vi "UHR-Fleezers Control (host) - 12.0.vi"() -> ()   [LabVIEW 2014] (continued)
            n2110 = property on="Trap Pos. FB ON" class="Bool (strict)"("Val(Sgnl)"=TRUE ("Value (Signaling)")) -> ()  [unwired: 2 in, 2 out]
            n2111 = Wait (ms)(milliseconds to wait=u32 250) -> ()  [unwired: 1 out]
          }
          frame #5 {
            n2112 = case shown="\"1\"" "Remove Action Offset Dropdown" {
              tunnel: TRUE ("Value (Signaling)") -> [w3020 w3028 w3036]
              frame "1" {
                n2113 = flat-sequence {
                  tunnel: w3020 -> [w3027]
                  frame #0 {
                    n2114 = local read "factor"() -> (w3022:dbl)
                    n2115 = Greater Than 0?(x=w3022) -> (x > 0?=w3026:bool)
                    n2116 = Select(t=1.0, s=w3026, f=-1.0) -> (s? t:f=w3023:dbl)
                    n2117 = Multiply(x=w3023, y=w3022) -> (x*y=w3021:dbl)
                    n2118 = local write "factor"(w3021) -> ()
                  }
                  frame #1 {
                    n2119 = property on="Remove Offset to factor" class="Bool (strict)"("Val(Sgnl)"=w3027) -> ()  [unwired: 2 in, 2 out]
                  }
                }
              }
              frame "2" {
                n2120 = flat-sequence {
                  tunnel: w3028 -> [w3035]
                  frame #0 {
                    n2121 = local read "factor"() -> (w3029:dbl)
                    n2122 = Greater Than 0?(x=w3029) -> (x > 0?=w3034:bool)
                    n2123 = Select(t=-1.0, s=w3034, f=1.0) -> (s? t:f=w3032:dbl)
                    n2124 = Multiply(x=w3029, y=w3032) -> (x*y=w3031:dbl)
                    n2125 = local write "factor"(w3031) -> ()
                  }
                  frame #1 {
                    n2126 = property on="Remove Offset to factor" class="Bool (strict)"("Val(Sgnl)"=w3035) -> ()  [unwired: 2 in, 2 out]
                  }
                }
              }
              frame "0", Default {
                n2127 = property on="Remove Action Offset" class="Bool (strict)"("Val(Sgnl)"=w3036) -> ()  [unwired: 2 in, 2 out]
              }
            }
            n2128 = case shown="False" "Trap Trig Fl." {
              frame False {
                n2129 = case shown="True" "Green ON after FB ON?" {
                  selector: "Green ON after FB ON?" -> [_ w3038]
                  frame False {
                  }
                  frame True {
                    n2130 = property on="Green ON/Interlacing" class="Bool (strict)"("Val(Sgnl)"=w3038) -> ()  [unwired: 2 in, 2 out]
                  }
                }
              }
              frame True {
              }
            }
            n2131 = Wait (ms)(milliseconds to wait=u32 250) -> ()  [unwired: 1 out]
          }
          frame #6 {
            n2132 = property on="Start Saving" class="Bool (strict)"("Val(Sgnl)"=TRUE ("Value (Signaling)")) -> ()  [unwired: 2 in, 2 out]
            n2133 = Wait (ms)(milliseconds to wait=u32 5000) -> ()  [unwired: 1 out]
          }
          frame #7 {
            w3042 = TRUE ("Value (Signaling)")
            n2134 = property on="Rem fb disp offset" class="Bool (strict)"("Val(Sgnl)"=w3042) -> ()  [unwired: 2 in, 2 out]
            n2135 = property on="Remove Offset" class="Bool (strict)"("Val(Sgnl)"=w3042) -> ()  [unwired: 2 in, 2 out]
            n2136 = Wait (ms)(milliseconds to wait=u32 100) -> ()  [unwired: 1 out]
          }
          frame #8 {
            n2137 = case shown="True" w3045 {
              frame False {
              }
              frame True {
                n2138 = local write "Trap Trig. Fl."(TRUE ("Value (Signaling)")) -> ()
              }
            }
          }
          frame #9 {
            n2139 = local read "Tether"() -> (w3048:bool)
            n2140 = And(x="Start dipping after?", y=w3048) -> (x .and. y?=w3047:bool)
            n2141 = case shown="True" w3047 {
              frame False {
              }
              frame True {
                n2142 = flat-sequence {
                  frame #0 {
                    n2143 = Multiply(x="Delay before dipping (s)", y=1000.0) -> (x*y=w3051:dbl)
                    n2144 = Wait (ms)(milliseconds to wait=w3051) -> ()  [unwired: 1 out]
                  }
                  frame #1 {
                    n2145 = property on="Dip for Protein" class="Bool (strict)"("Val(Sgnl)"=TRUE ("Value (Signaling)")) -> ()  [unwired: 2 in, 2 out]
                    n2146 = local write "Scripts"(T35."Dipping") -> ()
                  }
                }
              }
            }
          }
        }
      }
      event "Rupture Script": Value Change {
        n2147 = event-data() -> ()  [unwired: 1 in, 5 out]
        n2148 = local write "Rupture Script"(FALSE ("Rupture Script")) -> ()
        n2149 = flat-sequence {
          frame #0 {
            w3057 = TRUE
            w3062 = FALSE
            # "Number 6 for now is the\nrupture-experiment\nparameters."
            n2150 = local read "Starting Trap D (MHz)"() -> (w3063:dbl)
            n2151 = local write "Restart DMA? (AOD)"(w3062) -> ()
            n2152 = Replace Array Subset(array=u32[] [0] ("Index Values"), new element=6, index=0) -> (w3058:u32[])
            n2153 = local write "Save scans"(w3062) -> ()
            n2154 = property on="Trap D (MHz)" class="DigNum (strict)"("Val(Sgnl)"=w3063) -> ()  [unwired: 2 in, 2 out]
            n2155 = property on="Saved AOD Raster Scan Parameter Sets" class="Arr (strict)"("Index Values"=w3058) -> ()  [unwired: 2 in, 2 out]
            n2156 = property on="Start Saving" class="Bool (strict)"("Val(Sgnl)"=w3057) -> ()  [unwired: 2 in, 2 out]
            n2157 = property on="Green ON/Interlacing" class="Bool (strict)"("Val(Sgnl)"=w3057) -> ()  [unwired: 2 in, 2 out]
          }
          frame #1 {
            n2158 = property on="Load parameters" class="Bool (strict)"("Val(Sgnl)"=TRUE ("Value (Signaling)")) -> ()  [unwired: 2 in, 2 out]
          }
        }
      }
      event "Fixed Traps Script": Value Change {
        n2159 = event-data() -> ()  [unwired: 1 in, 5 out]
        n2160 = local write "Fixed Traps Script"(FALSE ("Fixed Traps Data\nScript")) -> ()
        n2161 = flat-sequence {
          frame #0 {
            n2162 = case shown="True" "Green ON" {
              frame False {
              }
              frame True {
                n2163 = property on="Green ON/Interlacing" class="Bool (strict)"("Val(Sgnl)"=TRUE) -> ()  [unwired: 2 in, 2 out]
              }
            }
            n2164 = local write "Offset (nm)"(0.0 ("Offset (nm)")) -> ()
            n2165 = property on="Sample Channel\nFlow" class="Bool (strict)"("Val(Sgnl)"=FALSE ("Value (Signaling)")) -> ()  [unwired: 2 in, 2 out]
            n2166 = property on="Trap D (MHz)" class="DigNum (strict)"("Val(Sgnl)"="Fixed Traps Trap Delta (MHz)") -> ()  [unwired: 2 in, 2 out]
          }
          frame #1 {
            n2167 = Wait (ms)(milliseconds to wait=u32 1000) -> ()  [unwired: 1 out]
          }
          frame #2 {
            n2168 = local write "Start Saving"(TRUE ("Start Saving")) -> ()
          }
          frame #3 {
            n2169 = local read "Bead Sep. Int. Time (s)"() -> (w3073:dbl)
            n2170 = Multiply(x=w3073, y=1000.0) -> (x*y=w3075:dbl)
            n2171 = Wait (ms)(milliseconds to wait=w3075) -> ()  [unwired: 1 out]
          }
          frame #4 {
            n2172 = property on="Remove Offset" class="Bool (strict)"("Val(Sgnl)"=TRUE ("Value (Signaling)")) -> ()  [unwired: 2 in, 2 out]
          }
          frame #5 {
            n2173 = property on="Dip for Protein" class="Bool (strict)"("Val(Sgnl)"="Start dipping after?") -> ()  [unwired: 2 in, 2 out]
          }
        }
      }
      event "Got DNA bead": Value Change {
        n2174 = event-data() -> ()  [unwired: 1 in, 5 out]
        n2175 = flat-sequence {
          frame #0 {
            w3079 = FALSE ("Key Focus")
            n2176 = local read "Daq spot flow on"() -> (w3080:bool)
            n2177 = case shown="True" w3080 {
              frame False {
              }
              frame True {
                n2178 = property on="Sample Channel\nFlow" class="Bool (strict)"("Val(Sgnl)"=TRUE ("Value (Signaling)")) -> ()  [unwired: 2 in, 2 out]
              }
            }
            n2179 = local write "Got DNA bead"(w3079) -> ()
            n2180 = property on="Got DNA bead" class="Bool (strict)"("Key Focus"=w3079) -> ()  [unwired: 2 in, 2 out]
          }
          frame #1 {
            n2181 = property on="Inject Pump 1" class="Bool (strict)"("Val(Sgnl)"=FALSE ("Value (Signaling)")) -> ()  [unwired: 2 in, 2 out]
          }
          frame #2 {
            n2182 = property on="Cal/Data Acq. Spot" class="Bool (strict)"("Val(Sgnl)"=TRUE ("Value (Signaling)")) -> ()  [unwired: 2 in, 2 out]
          }
        }
      }
      event "Take Stepping Data": Value Change {
        n2183 = event-data() -> ()  [unwired: 1 in, 5 out]
        n2184 = local read "Save ave N"() -> (w3092:dbl)
        n2185 = flat-sequence {
          tunnel: w3092 -> [w3094]
          tunnel: [w3094] -> w3087
          tunnel: [w3096] -> w3088
          tunnel: w3087 -> [w3096]
          tunnel: [w3098] -> w3089
          tunnel: w3088 -> [w3098]
          tunnel: [w3101] -> w3090
          tunnel: w3089 -> [w3101]
          tunnel: [w3103] -> w3091
          tunnel: w3090 -> [w3103]
          tunnel: [w3105] -> w3085
          tunnel: w3091 -> [w3105]
          tunnel: w3085 -> [w3108]
          tunnel: [w3108] -> w3084
          tunnel: w3084 -> [w3109]
          tunnel: [w3109] -> w3086
          tunnel: w3086 -> [w3115]
          frame #0 {
            n2186 = property on="Save ave N" class="DigNum (strict)"("Val(Sgnl)"="Save ave factor") -> ()  [unwired: 2 in, 2 out]
          }
          frame #1 {
            n2187 = Wait (ms)(milliseconds to wait=u32 100) -> ()  [unwired: 1 out]
          }
          frame #2 {
            n2188 = local read "Offset 2 Start (MHz)"() -> (w3100:dbl)
            n2189 = property on="Saved AOD Raster Scan Parameter Sets" class="Arr (strict)"("Index Values"=u32[] [2]) -> ()  [unwired: 2 in, 2 out]
            n2190 = property on="Trap D (MHz)" class="DigNum (strict)"("Val(Sgnl)"=w3100) -> ()  [unwired: 2 in, 2 out]
          }
          frame #3 {
            n2191 = property on="Load parameters" class="Bool (strict)"("Val(Sgnl)"=TRUE ("Value (Signaling)")) -> ()  [unwired: 2 in, 2 out]
          }
          frame #4 {
            n2192 = Wait (ms)(milliseconds to wait=u32 100) -> ()  [unwired: 1 out]
          }
          frame #5 {
            n2193 = property on="Trap Raster Scan" class="Bool (strict)"("Val(Sgnl)"=TRUE ("Value (Signaling)")) -> ()  [unwired: 2 in, 2 out]
          }
          frame #6 {
            n2194 = Wait (ms)(milliseconds to wait=u32 1000) -> ()  [unwired: 1 out]
          }
          frame #7 {
            n2195 = while {
              stop <- w3112 stop-if-true
              n2196 = local read "Raster Scanning..."() -> (w3114:bool)
              n2197 = local read "Saving..."() -> (w3113:bool)
              n2198 = Not(x=w3113) -> (.not. x?=w3110:bool)
              n2199 = Not(x=w3114) -> (.not. x?=w3111:bool)
              n2200 = And(x=w3111, y=w3110) -> (x .and. y?=w3112:bool)
            }
          }
          frame #8 {
            n2201 = property on="Save ave N" class="DigNum (strict)"("Val(Sgnl)"=w3115) -> ()  [unwired: 2 in, 2 out]
          }
        }
      }
      event "Step Size (nm)": Value Change {
        n2202 = event-data() -> ()  [unwired: 1 in, 5 out]
        n2203 = flat-sequence {
          frame #0 {
            n2204 = property on="Saved AOD Raster Scan Parameter Sets" class="Arr (strict)"("Index Values"=u32[] [1]) -> ()  [unwired: 2 in, 2 out]
          }
          frame #1 {
            n2205 = Multiply(x="N Steps", y="Step Size (nm)") -> (x*y=w3117:dbl)
            n2206 = property on="Scan Speed AOD (nm/s) 2" class="DigNum (strict)"("Value"="Step Size (nm)") -> ()  [unwired: 2 in, 2 out]
            n2207 = property on="Step Size AOD (nm) 2" class="DigNum (strict)"("Value"="Step Size (nm)") -> ()  [unwired: 2 in, 2 out]
            n2208 = property on="Scan Range AOD (nm) 2" class="DigNum (strict)"("Value"=w3117) -> ()  [unwired: 2 in, 2 out]
          }
        }
      }
      event "Take Detection Laser\nImage": Value Change {
        n2209 = event-data() -> ()  [unwired: 1 in, 5 out]
        n2210 = flat-sequence {
          tunnel: [w3145] -> w3135
          tunnel: [w3144] -> w3128
          tunnel: [w3143] -> w3120
          tunnel: [w3148] -> w3136
          tunnel: w3135 -> [w3148]
          tunnel: [w3147] -> w3129
          tunnel: w3128 -> [w3147]
          tunnel: [w3146] -> w3121
          tunnel: w3120 -> [w3146]
          tunnel: [w3152] -> w3137
          tunnel: w3136 -> [w3152]
          tunnel: [w3151] -> w3130
          tunnel: w3129 -> [w3151]
          tunnel: [w3150] -> w3122
          tunnel: w3121 -> [w3150]
          tunnel: [w3158] -> w3138
          tunnel: w3137 -> [w3158]
          tunnel: [w3157] -> w3131
          tunnel: w3130 -> [w3157]
          tunnel: [w3156] -> w3123
          tunnel: w3122 -> [w3156]
          tunnel: [w3162] -> w3139
          tunnel: w3138 -> [w3162]
          tunnel: [w3161] -> w3132
          tunnel: w3131 -> [w3161]
          tunnel: [w3160] -> w3124
          tunnel: w3123 -> [w3160]
          tunnel: [w3166] -> w3140
          tunnel: w3139 -> [w3166]
          tunnel: [w3165] -> w3133
          tunnel: w3132 -> [w3165]
          tunnel: [w3164] -> w3125
          tunnel: w3124 -> [w3164]
          tunnel: [w3170] -> w3141
          tunnel: w3140 -> [w3170]
          tunnel: [w3169] -> w3134
          tunnel: w3133 -> [w3169]
          tunnel: [w3168] -> w3126
          tunnel: w3125 -> [w3168]
          tunnel: w3141 -> [w3176]
          tunnel: w3134 -> [w3175]
          tunnel: [w3173] -> w3127
          tunnel: w3126 -> [w3173]
          tunnel: w3127 -> [w3177]
          frame #0 {
            n2211 = local read "Laser interlacing mode (all lasers)"() -> (w3144:enum32{"Laser ON", "Laser OFF", "Interlace"})
            n2212 = local read "Green ON/Interlacing"() -> (w3145:bool)
            n2213 = local read "Green FB On/Off"() -> (w3143:bool)
          }
          frame #1 {
            n2214 = property on="Green FB On/Off" class="Bool (strict)"("Val(Sgnl)"=FALSE ("Value (Signaling)")) -> ()  [unwired: 2 in, 2 out]
          }
          frame #2 {
            n2215 = property on="Green ON/Interlacing" class="Bool (strict)"("Val(Sgnl)"=TRUE ("Value (Signaling)")) -> ()  [unwired: 2 in, 2 out]
            n2216 = property on="Flip Green Filter" class="Bool (strict)"("Val(Sgnl)"=TRUE ("Value (Signaling)")) -> ()  [unwired: 2 in, 2 out]
            n2217 = property on="Laser interlacing mode (all lasers)" class="RadioBtnsControl (strict)"("Val(Sgnl)"=enum32{"Laser ON", "Laser OFF", "Interlace"}."Laser ON" ("Value (Signaling)")) -> ()  [unwired: 2 in, 2 out]
          }
          frame #3 {
            n2218 = Wait (ms)(milliseconds to wait=u32 500) -> ()  [unwired: 1 out]
          }
          frame #4 {
            n2219 = property on="Confocal\nImage" class="Bool (strict)"("Val(Sgnl)"=TRUE ("Value (Signaling)")) -> ()  [unwired: 2 in, 2 out]
          }
          frame #5 {
            n2220 = Wait (ms)(milliseconds to wait=u32 2000) -> ()  [unwired: 1 out]
          }
          frame #6 {
            n2221 = while {
              stop <- w3171 stop-if-true
              n2222 = local read "Saving..."() -> (w3172:bool)
              n2223 = Not(x=w3172) -> (.not. x?=w3171:bool)
            }
          }
          frame #7 {
            n2224 = property on="Flip Green Filter" class="Bool (strict)"("Val(Sgnl)"=TRUE ("Value (Signaling)")) -> ()  [unwired: 2 in, 2 out]
            n2225 = property on="Green ON/Interlacing" class="Bool (strict)"("Val(Sgnl)"=w3176) -> ()  [unwired: 2 in, 2 out]
            n2226 = property on="Laser interlacing mode (all lasers)" class="RadioBtnsControl (strict)"("Val(Sgnl)"=w3175) -> ()  [unwired: 2 in, 2 out]
          }
          frame #8 {
            n2227 = property on="Green FB On/Off" class="Bool (strict)"("Val(Sgnl)"=w3177) -> ()  [unwired: 2 in, 2 out]
          }
        }
      }
      event "Stop All": Value Change {
        n2228 = event-data() -> ()  [unwired: 1 in, 5 out]
        n2229 = local read "Stop All"() -> (w3178:bool)
      }
    }
    n2230 = node-c288() -> ()  [unwired: 1 in, 1 out]
  }
  n2231 = node-c288() -> (w139:T26)  [unwired: 4 out]
  n2232 = timed-loop "Mouse control: trap position (AOM deflection), set confocal spot from image" {
    tunnel: [w3180] -> w224
    tunnel: w51 -> [w3179]
    timing: w139 -> [_]
    timing-out: [_] -> w138
    stop <- w3180 stop-if-true
    n2233 = node-c288() -> ()  [unwired: 2 out]
    n2234 = event shown="[0] \"Pane\": Mouse Down" {
      selector: _ -> [_ _]
      dyn-events: _ -> [_ _]
      timeout: _ -> [_ _]
      tunnel: w3179 -> [w3183 _]
      event Mouse Down {
        n2235 = event-data() -> ("Time"=w3185:u32, "Coords"=w3184:T7, "Button"=w3186:u16)  [unwired: 6 out]
        n2236 = case shown="1" w3186 {
          tunnel: w3185 -> [_ _ w3325]
          tunnel: w3184 -> [_ w3191 w3323]
          tunnel: w3183 -> [_ _ w3321]
          frame 0, Default {
          }
          frame 1 {
            n2237 = property on="APD 2" class="ImageControl"() -> ("Displayed Image Position"=w3205:cluster{"Left":i32, "Top":i32})  [unwired: 2 in, 2 out]
            n2238 = control-ref of="Primary Video Display"() -> (w3198:refnum<vi>)
            n2239 = property on="APD 1" class="ImageControl"() -> ("Displayed Image Position"=w3234:cluster{"Left":i32, "Top":i32})  [unwired: 2 in, 2 out]
            n2240 = property on="Detection Laser X" class="ImageControl"() -> ("Displayed Image Position"=w3231:cluster{"Left":i32, "Top":i32})  [unwired: 2 in, 2 out]
            n2241 = property on="Detection Laser Y" class="ImageControl"() -> ("Displayed Image Position"=w3230:cluster{"Left":i32, "Top":i32})  [unwired: 2 in, 2 out]
            n2242 = property on="APD 2" class="ImageControl"() -> ("Displayed Image Size"=w3204:cluster{"Width":u32, "Height":u32})  [unwired: 2 in, 2 out]
            n2243 = property on="APD 1" class="ImageControl"() -> ("Displayed Image Size"=w3232:cluster{"Width":u32, "Height":u32})  [unwired: 2 in, 2 out]
            n2244 = property on="Detection Laser X" class="ImageControl"() -> ("Displayed Image Size"=w3233:cluster{"Width":u32, "Height":u32})  [unwired: 2 in, 2 out]
            n2245 = property on="Detection Laser Y" class="ImageControl"() -> ("Displayed Image Size"=w3229:cluster{"Width":u32, "Height":u32})  [unwired: 2 in, 2 out]
            n2246 = property class="ImageControl"(reference=w3198) -> ("Displayed Image Position"=w3196:cluster{"Left":i32, "Top":i32})  [unwired: 1 in, 2 out]
            n2247 = property class="ImageControl"(reference=w3198) -> ("Displayed Image Size"=w3197:cluster{"Width":u32, "Height":u32})  [unwired: 1 in, 2 out]
            n2248 = Unbundle By Name(w3204) -> ("Width"=w3201:u32, "Height"=w3200:u32)
            n2249 = Unbundle By Name(w3205) -> ("Left"=w3203:i32, "Top"=w3202:i32)
            n2250 = Unbundle By Name(w3232) -> ("Width"=w3226:u32, "Height"=w3225:u32)
            n2251 = Unbundle By Name(w3233) -> ("Width"=w3222:u32, "Height"=w3221:u32)
            n2252 = Unbundle By Name(w3229) -> ("Width"=w3218:u32, "Height"=w3217:u32)
            n2253 = Unbundle By Name(w3234) -> ("Left"=w3228:i32, "Top"=w3227:i32)
            n2254 = Unbundle By Name(w3231) -> ("Left"=w3224:i32, "Top"=w3223:i32)
            n2255 = Unbundle By Name(w3230) -> ("Left"=w3220:i32, "Top"=w3219:i32)
            n2256 = Bundle("Left"=w3203, "Top"=w3202, "Width"=w3201, "Height"=w3200) -> (w3199:T36)  [unwired: 1 in]
            n2257 = Bundle("Left"=w3228, "Top"=w3227, "Width"=w3226, "Height"=w3225) -> (w3216:T36)  [unwired: 1 in]
            n2258 = Bundle("Left"=w3224, "Top"=w3223, "Width"=w3222, "Height"=w3221) -> (w3215:T36)  [unwired: 1 in]
            n2259 = Bundle("Left"=w3220, "Top"=w3219, "Width"=w3218, "Height"=w3217) -> (w3214:T36)  [unwired: 1 in]
            n2260 = Unbundle By Name(w3197) -> ("Width"=w3193:u32, "Height"=w3192:u32)
            n2261 = Unbundle By Name(w3196) -> ("Left"=w3195:i32, "Top"=w3194:i32)
            n2262 = Build Cluster Array(w3199, w3216, w3215, w3214) -> (w3213:T37)
            n2263 = Bundle("Left"=w3195, "Top"=w3194, "Width"=w3193, "Height"=w3192) -> (w3188:T36)  [unwired: 1 in]
            n2264 = for {
              tunnel: w3191 -> [w3267]
              tunnel: w3213 -> [w3268] mode=indexing
              shift-right: [w3265] -> w3211
              shift-left: TRUE -> [w3266]
              shift-right: [w3264] -> w3209
              shift-left: _ -> [w3260]
              shift-right: [w3263] -> w3208
              shift-left: _ -> [w3259]
              shift-right: [w3262] -> w3207
              shift-left: _ -> [w3258]
              shift-right: [w3261] -> w3206
              shift-left: _ -> [w3257]
              n2265 = case shown="True" w3266 {
                selector: w3266 -> [w3273 _]
                tunnel: w3268 -> [_ w3282]
                tunnel: w3267 -> [_ w3280]
                tunnel: [w3273 w3278] -> w3265
                tunnel: [w3272 w3277] -> w3264
                tunnel: [w3271 w3276] -> w3263
                tunnel: [w3270 w3275] -> w3262
                tunnel: [w3269 w3274] -> w3261
                tunnel: w3260 -> [w3272 _]
                tunnel: w3259 -> [w3271 _]
                tunnel: w3258 -> [w3270 _]
                tunnel: w3257 -> [w3269 _]
                frame False {
                }
                frame True {
                  n2266 = Unbundle(w3282) -> (w3281:T36)
                  n2267 = call "isclickinwindow.vi"("Image Param"=w3281, "Point32"=w3280) -> ("4 Y"=w3274:i32, "3 Height"=w3275:i32, "2 X"=w3276:i32, "1 Width"=w3277:i32, "In image?"=w3279:bool)  [unwired: 1 in]
                  n2268 = Not(x=w3279) -> (.not. x?=w3278:bool)
                }
              }
            }
            n2269 = call "isclickinwindow.vi"("Image Param"=w3188, "Point32"=w3191) -> ("4 Y"=w3189:i32, "2 X"=w3190:i32, "In image?"=w3187:bool)  [unwired: 1 in, 2 out]
            n2270 = case shown="True" w3187 {
              tunnel: w3190 -> [_ w3238]
              tunnel: w3189 -> [_ w3241]
              frame False {
              }
              frame True {
                w3250 = 2
                n2271 = Subtract(x=480, y=w3241) -> (x-y=w3240:i32)
                n2272 = Unbundle("Target size") -> ("Width"=w3251:dbl, "Height"=w3249:dbl)
                n2273 = Subtract(x=w3238, y=2) -> (x-y=w3237:i32)
                n2274 = Divide(x=w3249, y=w3250) -> (x/y=w3247:dbl)
                n2275 = Divide(x=w3251, y=w3250) -> (x/y=w3248:dbl)
                n2276 = Subtract(x=w3237, y=w3248) -> (x-y=w3246:dbl)
                n2277 = Add(x=w3237, y=w3248) -> (x+y=w3244:dbl)
                n2278 = Subtract(x=w3240, y=w3247) -> (x-y=w3245:dbl)
                n2279 = Add(x=w3240, y=w3247) -> (x+y=w3243:dbl)
                n2280 = Bundle(w3237, w3240) -> (w3253:cluster{i32, i32})  [unwired: 1 in]
                n2281 = Bundle(w3246, w3245, w3244, w3243) -> (w3235:cluster{dbl, dbl, dbl, dbl})  [unwired: 1 in]
                n2282 = case shown="True" "Set target" {
                  tunnel: w3253 -> [_ w3256]
                  tunnel: w3235 -> [_ w3254]
                  frame False {
                  }
                  frame True {
                    n2283 = local write "Target coordinates"(w3254) -> ()
                    n2284 = local write "Set target"(FALSE ("Set target")) -> ()
                    "Video coordinates" <- w3256
                  }
                }
              }
            }
            n2285 = Not(x=w3211) -> (.not. x?=w3210:bool)
            n2286 = case shown="True" w3210 {
              tunnel: w3208 -> [_ w3296]
              tunnel: w3206 -> [_ w3295]
              tunnel: w3209 -> [_ w3294]
              tunnel: w3207 -> [_ w3293]
              frame False {
              }
              frame True {
                w3283 = FALSE ("Get Point")
                n2287 = local read "Scan lines (y)"() -> (w3298:u64)
                n2288 = disable-structure shown="Disabled" {
                  frame Disabled {
                  }
                  frame Enabled {
                  }
                }
                n2289 = local read "Actual MCL Inc (V)"() -> (w3292:dbl)
                n2290 = local read "Scan steps (MCL)"() -> (w3297:u64)
                n2291 = Divide "Y Pix/step"(x=w3293, y=w3298) -> (x/y=w3305:dbl)
                n2292 = Divide "Y V/pix"(x=w3292, y=w3305) -> (x/y=w3304:dbl)
                n2293 = Divide "Y half step offset"(x=w3292, y=2.0) -> (x/y=w3306:dbl)
                n2294 = Divide "X pix/step"(x=w3294, y=w3297) -> (x/y=w3303:dbl)
                n2295 = Negate(x=w3306) -> (-x=w3307:dbl)
                n2296 = local read "Initial Y"() -> (w3313:dbl)
                n2297 = Multiply(x=w3295, y=w3304) -> (x*y=w3314:dbl)
                n2298 = Divide "X half step offset"(x=w3292, y=2.0) -> (x/y=w3300:dbl)
                n2299 = Divide "X V/pix"(x=w3292, y=w3303) -> (x/y=w3302:dbl)
                n2300 = Multiply(x=w3292, y=w3297) -> (x*y=w3309:dbl)
                n2301 = Compound Arithmetic op=ADD(w3307, w3314, w3313) -> (w3284:dbl)
                "Pointer Y (V)" <- w3284
                n2302 = Multiply(x=w3302, y=w3296) -> (x*y=w3311:dbl)
                n2303 = Negate(x=w3300) -> (-x=w3299:dbl)
                n2304 = local read "Initial X"() -> (w3312:dbl)
                n2305 = Negate(x=w3311) -> (-x=w3310:dbl)
                n2306 = Compound Arithmetic op=ADD(w3299, w3309, w3312, w3310) -> (w3285:dbl)
                "Pointer X (V)" <- w3285
                n2307 = case shown="True" "Set High F Confocal Spot (X-Y)" {
                  tunnel: w3285 -> [_ w3315]
                  tunnel: w3284 -> [_ w3316]
                  frame False {
                  }
                  frame True {
                    "Confocal Y 2 (V)" <- w3316
                    "Confocal X 2 (V)" <- w3315
                  }
                }
                n2308 = Or(x="Set X Only", y="Set Confocal Spot (X-Y)") -> (x .or. y?=w3288:bool)
                n2309 = Or(x="Set Confocal Spot (X-Y)", y="Set Y Only") -> (x .or. y?=w3287:bool)
                n2310 = case shown="True" w3288 {
                  tunnel: w3285 -> [_ w3317]
                  frame False {
                  }
                  frame True {
                    n2311 = property on="AO2" class="Slide (strict)"("Val(Sgnl)"=w3317) -> ()  [unwired: 2 in, 2 out]
                    "Confocal X 1 (V)" <- w3317
                  }
                }
                n2312 = case shown="True" w3287 {
                  tunnel: w3284 -> [_ w3318]
                  frame False {
                  }
                  frame True {
                    n2313 = property on="AO1" class="Slide (strict)"("Val(Sgnl)"=w3318) -> ()  [unwired: 2 in, 2 out]
                    "Confocal Y 1 (V)" <- w3318
                  }
                }
                n2314 = local write "Set High F Confocal Spot (X-Y)"(w3283) -> ()
                n2315 = local write "Set Confocal Spot (X-Y)"(w3283) -> ()
                n2316 = local write "Set X Only"(w3283) -> ()
                n2317 = local write "Set Y Only"(w3283) -> ()
              }
            }
          }
          frame 3 {
            n2318 = local read "BD 2 Frequency 1 (MHz)"() -> (w3319:dbl)
            n2319 = local read "BD 1 Frequency 1 (MHz)"() -> (w3320:dbl)
            n2320 = local write "Manipulating Trap"(TRUE ("Manipulating Trap")) -> ()
            n2321 = local write "Coords"(T7 {"Horizontal"=0, "Vertical"=0} ("Coords")) -> ()
            n2322 = while {
              tunnel: w3325 -> [w3330]
              tunnel: w3323 -> [w3329]
              tunnel: w3321 -> [w3328]
              tunnel: w3320 -> [w3327]
              tunnel: w3319 -> [w3326]
              stop <- w3331 stop-if-true
              n2323 = event shown="[0] \"Pane\": Mouse Move" {
                selector: _ -> [_ _]
                dyn-events: _ -> [_ _]
                timeout: _ -> [_ _]
                tunnel: ["Force Manip Abort" w3395] -> w3331
                tunnel: w3330 -> [w3338 _]
                tunnel: w3329 -> [w3336 _]
                tunnel: w3328 -> [w3335 _]
                tunnel: w3327 -> [w3334 _]
                tunnel: w3326 -> [w3333 _]
                event Mouse Move {
                  n2324 = event-data() -> ("Time"=w3339:u32, "Coords"=w3340:T7)  [unwired: 3 out]
                  n2325 = Less?(x=w3339, y=w3338) -> (x < y?=w3337:bool)
                  n2326 = case "Makes sure old motion events prior to mouse click aren't used" shown="False" w3337 {
                    tunnel: w3340 -> [w3382 _]
                    tunnel: w3336 -> [w3383 _]
                    tunnel: w3335 -> [w3360 _]
                    tunnel: w3334 -> [w3356 _]
                    tunnel: w3333 -> [w3355 _]
                    frame False {
                      n2327 = Subtract(x=w3382, y=w3383) -> (x-y=w3381:T7)
                      "Coords" <- w3381
                      n2328 = local read "Y RF Frequency Limits (MHz)"() -> (w3341:T17)
                      n2329 = To Double Precision Float(number=w3381) -> (double precision float=w3380:cluster{"Horizontal":dbl, "Vertical":dbl})
                      n2330 = Multiply(x=cluster{"Horizontal":dbl, "Vertical":dbl} {"Horizontal"=-1.0, "Vertical"=1.0}, y="Manipulation Scaling") -> (x*y=w3376:cluster{"Horizontal":dbl, "Vertical":dbl})
                      n2331 = local read "X RF Frequency Limits (MHz)"() -> (w3342:T17)
                      n2332 = Multiply(x=w3380, y=w3376) -> (x*y=w3378:cluster{"Horizontal":dbl, "Vertical":dbl})
                      n2333 = Unbundle By Name(w3378) -> ("Horizontal"=w3373:dbl, "Vertical"=w3377:dbl)
                      n2334 = Unbundle By Name(w3341) -> ("Maximum"=w3344:dbl, "Minimum"=w3343:dbl)
                      n2335 = Boolean To (0,1)(Boolean="Manip. X?") -> (0, 1=w3371:i16)
                      n2336 = Boolean To (0,1)(Boolean="Manip. Y?") -> (0, 1=w3368:i16)
                      n2337 = local read "BD 1 Frequency 2 (MHz)"() -> (w3358:dbl)
                      n2338 = Multiply(x=w3377, y=w3368) -> (x*y=w3370:dbl)
                      n2339 = Multiply(x=w3371, y=w3373) -> (x*y=w3374:dbl)
                      n2340 = local read "BD 2 Frequency 2 (MHz)"() -> (w3357:dbl)
                      n2341 = Unbundle By Name(w3342) -> ("Maximum"=w3346:dbl, "Minimum"=w3345:dbl)
                      n2342 = Add(x=w3355, y=w3370) -> (x+y=w3348:dbl)
                      n2343 = Add(x=w3356, y=w3374) -> (x+y=w3350:dbl)
                      n2344 = In Range and Coerce(upper limit=w3346, x=w3350, lower limit=w3345) -> (coerced(x)=w3349:dbl)  [unwired: 1 out]
                      n2345 = In Range and Coerce(upper limit=w3344, x=w3348, lower limit=w3343) -> (coerced(x)=w3347:dbl)  [unwired: 1 out]
                      n2346 = Subtract(x=w3349, y=w3358) -> (x-y=w3367:dbl)
                      n2347 = Subtract(x=w3347, y=w3357) -> (x-y=w3366:dbl)
                      n2348 = Square(x=w3367) -> (x^2=w3365:dbl)
                      n2349 = Square(x=w3366) -> (x^2=w3364:dbl)
                      n2350 = Add(x=w3365, y=w3364) -> (x+y=w3363:dbl)
                      n2351 = Square Root(x=w3363) -> (sqrt(x)=w3359:dbl)
                      n2352 = In Range and Coerce(upper limit="Limit Max (MHz)", x=w3359, lower limit="Limit Min (MHz)") -> (In Range?=w3352:bool)  [unwired: 1 out]
                      n2353 = Not(x="Limits Enable") -> (.not. x?=w3351:bool)
                      n2354 = Or(x=w3352, y=w3351) -> (x .or. y?=w3353:bool)
                      n2355 = case shown="True" w3353 {
                        tunnel: w3360 -> [_ w3393]
                        tunnel: w3359 -> [_ w3384]
                        tunnel: w3349 -> [_ w3391]
                        tunnel: w3358 -> [_ w3390]
                        tunnel: w3347 -> [_ w3389]
                        tunnel: w3357 -> [_ w3388]
                        tunnel: w3342 -> [_ w3386]
                        tunnel: w3341 -> [_ w3385]
                        frame False {
                        }
                        frame True {
                          n2356 = local read "BD 1 Frequency 3 (MHz)"() -> (w3392:dbl)
                          n2357 = local read "BD 2 Frequency 3 (MHz)"() -> (w3387:dbl)
                          n2358 = local write "Trap D (MHz)"(w3384) -> ()
                          n2359 = call "set RF board frequency - interlace.vi"("Board 2 Frequency Limits"=w3385, "Board 1 Frequency Limits"=w3386, "FPGA VI Reference In"=w3393, "Board 2 Frequency 3 (MHz)"=w3387, "Board 1 Frequency 3 (MHz)"=w3392, "Board 2 Frequency 2 (MHz)"=w3388, "Board 2 Frequency 1 (MHz)"=w3389, "Board 1 Frequency 2 (MHz)"=w3390, "Board 1 Frequency 1  (MHz)"=w3391) -> ()  [unwired: 1 in, 2 out]
                          n2360 = local write "BD 2 Frequency 1 (MHz)"(w3389) -> ()
                          n2361 = local write "BD 1 Frequency 1 (MHz)"(w3391) -> ()
                        }
                      }
                    }
                    frame True {
                    }
                  }
                }
                event Mouse Up {
                  n2362 = event-data() -> ("Button"=w3394:u16)  [unwired: 8 out]
                  n2363 = case shown="3" w3394 {
                    tunnel: [FALSE TRUE] -> w3395
                    frame 0, Default {
                    }
                    frame 3 {
                      n2364 = local read "Trap D (MHz)"() -> (w3397:dbl)
                      n2365 = property on="Initial D (MHz)" class="DigNum (strict)"("Val(Sgnl)"=w3397) -> ()  [unwired: 2 in, 2 out]
                      n2366 = local write "Manipulating Trap"(FALSE ("Manipulating Trap")) -> ()
                    }
                  }
                }
              }
            }
          }
        }
      }
      event Mouse Move {
        n2367 = event-data() -> ()  [unwired: 6 out]
      }
    }
    n2368 = local read "Stop All"() -> (w3180:bool)
    n2369 = node-c288() -> ()  [unwired: 2 out]
  }
  n2370 = node-c288(w136) -> ()  [unwired: 1 out]
  n2371 = node-c288(w138) -> ()  [unwired: 1 out]
  n2372 = node-c288(w125) -> ()  [unwired: 1 out]
  n2373 = flat-sequence "Video" {
    tunnel: [w3408] -> w127
    tunnel: w127 -> [w3449]
    frame #0 {
      n2374 = while {
        stop <- w3401 continue-if-true
        n2375 = call "Close Video Capture.vi"() -> ("error code OUT"=w3403:i32)
        n2376 = Equal?(x=w3403, y=0) -> (x = y?=w3401:bool)
      }
      n2377 = local write "Stop All"(FALSE ("Stop All")) -> ()
    }
    frame #1 {
      n2378 = call "DMR_Init.vi"() -> ()  [unwired: 3 out]
    }
    frame #2 {
      # "Setting the destination format to Mono8 makes sure that the image can be displayed in the intensity plot."
      n2379 = call "DMR_GetDevice.vi"("search string IN"="DE019116701") -> ("device handle OUT"=w3426:i32)  [unwired: 4 in, 2 out]
      n2380 = call "DMR_OpenDevice.vi"("device handle IN"=w3426) -> ("driver handle OUT"=w3409:i32)  [unwired: 4 out]
      n2381 = call "DMR_FindList.vi"("flags IN"=u32 0 ("flags"), "list name IN"="" ("String"), "list type IN"=T38."camera descriptions", "driver handle IN"=w3409) -> ("list handle OUT"=w3412:i32)  [unwired: 2 out]
      n2382 = call "DMR_FindList.vi"("flags IN"=u32 0 ("flags"), "list name IN"="Base", "list type IN"=T38."setting", "driver handle IN"=w3409) -> ("list handle OUT"=w3410:i32)  [unwired: 2 out]
      n2383 = call "OBJ_GetHandle.vi"("object name IN"="VideoStandard", "list handle IN"=w3412) -> ("object handle OUT"=w3406:i32)  [unwired: 3 out]
      n2384 = call "OBJ_GetHandle.vi"("object name IN"="PixelFormat", "list handle IN"=w3410) -> ("object handle OUT"=w3420:i32)  [unwired: 3 out]
      n2385 = call "OBJ_SetS.vi"("value index IN"=0, "value IN"="NTSC M", "object handle IN"=w3406) -> ()  [unwired: 2 out]
      n2386 = call "OBJ_SetS.vi"("value index IN"=0, "value IN"="Mono8" ("value"), "object handle IN"=w3420) -> ()  [unwired: 2 out]
      n2387 = call "OBJ_GetHandle.vi"("object name IN"="VideoChannel", "list handle IN"=w3410) -> ("object handle OUT"=w3416:i32)  [unwired: 3 out]
      n2388 = while {
        tunnel: [w3431] -> w3408
        tunnel: w3409 -> [w3428]
        stop <- w3429 continue-if-true
        n2389 = call "DMR_ImageRequestSingle.vi"("request control IN"=0, "driver handle IN"=w3428) -> ("error code OUT"=w3430:i32, "driver handle OUT"=w3431:i32)  [unwired: 2 out]
        n2390 = Equal To 0?(x=w3430) -> (x = 0?=w3429:bool)
      }
      n2391 = call "OBJ_SetI.vi"("value index IN"=0, "value IN"=3 ("Video channel"), "object handle IN"=w3416) -> ()  [unwired: 2 out]
    }
    frame #3 {
      w3437 = T20 0 items=["Grayscale (U8)", "Grayscale (I16)", "Grayscale (SGL)", "Complex (CSG)", "RGB (U32)", "HSL (U32)", "RGB (U64)"] ("Image Type")
      w3445 = T20 0 items=["Grayscale (U8)", "Grayscale (I16)", "Grayscale (SGL)", "Complex (CSG)", "RGB (U32)", "HSL (U32)", "RGB (U64)"] ("Image Type")
      n2392 = for "Create Greyscale map" {
        N: 256 -> [_]
        tunnel: [w3451] -> w3434 mode=indexing
        workers-P: _ -> [_]
        i -> [w3454]
        n2393 = To Unsigned Byte Integer(number=w3454) -> (unsigned 8bit integer=w3450:u8)
        n2394 = Join Numbers(hi=w3450, lo=w3450) -> ((hi.lo)=w3453:u16)
        n2395 = Join Numbers(hi=w3450, lo=w3450) -> ((hi.lo)=w3452:u16)
        n2396 = Join Numbers(hi=w3453, lo=w3452) -> ((hi.lo)=w3451:u32)
      }
      n2397 = call "IMAQ Create"("Image Name"="Scaled video", "Image Type"=w3437) -> ("New Image"=w3436:T2)  [unwired: 2 in, 2 out]
      n2398 = call "IMAQ Create"("Image Name"="Main video", "Image Type"=w3445) -> ("New Image"=w3446:T2)  [unwired: 2 in, 2 out]
      n2399 = node-c288(0 ("Processor")) -> (w3444:T26)  [unwired: 3 out]
      n2400 = Initialize Array(u32 0 ("Window Number (0...15)"), 480 ("dimension size"), 640 ("dimension size")) -> (w3439:u32[][])
      n2401 = timed-loop {
        tunnel: w3449 -> [w3471]
        tunnel: [w3470] -> w3448
        tunnel: w3446 -> [w3469]
        timing: w3444 -> [_]
        timing-out: [_] -> w3443
        tunnel: w3439 -> [w3458]
        tunnel: w3436 -> [w3456]
        tunnel: w3434 -> [w3455]
        stop <- w3457 stop-if-true
        # "This block performs the \nactual image capture."
        n2402 = node-c288() -> ()  [unwired: 2 out]
        n2403 = local read "Stop All"() -> (w3457:bool)
        n2404 = Reciprocal(x="Video Capture Rate (Hz)") -> (1/x=w3461:dbl)
        n2405 = Multiply(x=w3461, y=1000.0) -> (x*y=w3459:dbl)
        n2406 = call "DMR_ImageRequestWaitFor.vi"("queue number IN"=0, "timeout(ms) IN"=500, "driver handle IN"=w3471) -> ("error code OUT"=w3475:i32, "request number OUT"=w3472:i32, "driver handle OUT"=w3473:i32)
        n2407 = feedback #1(T39 refnum ("Avi Refnum")) -> (w3463:T39)
        n2408 = case shown="True" "New Video File" {
          tunnel: [T39 refnum ("Avi Refnum") w3492] -> w3465
          tunnel: [FALSE TRUE] -> w3466
          tunnel: w3463 -> [_ w3488]
          frame False {
          }
          frame True {
            n2409 = call "Create new save file.vi"("Ext"=".avi" ("string"), "Index In"="Video Index") -> ("Path Out"=w3484:path, "Index Out"=w3485:dbl)  [unwired: 1 in]
            "Path Out" <- w3484
            n2410 = Not Equal?(x=w3488, y=T39 refnum ("Avi Refnum")) -> (x != y?=w3489:bool)
            n2411 = Increment(x=w3485) -> (x+1=w3494:dbl)
            n2412 = case shown="True" w3489 {
              tunnel: w3488 -> [_ w3495]
              frame False {
              }
              frame True {
                n2413 = call "IMAQ AVI Close"("Avi Refnum"=w3495) -> ()  [unwired: 1 in, 10 out]
              }
            }
            n2414 = local write "Video Index"(w3494) -> ()
            n2415 = call "IMAQ AVI Create"("Frames Per Second"=u32 30, "AVI Path"=w3484) -> ("Avi Refnum"=w3492:T39)  [unwired: 5 in, 4 out]
          }
        }
        n2416 = Equal To 0?(x=w3475) -> (x = 0?=w3474:bool)
        n2417 = Select(t=w3465, s=w3466, f=w3463) -> (s? t:f=w3464:T39)
        n2418 = feedback-in #1(w3464) -> ()
        n2419 = case shown="True" w3474 {
          tunnel: w3473 -> [w3496 w3523]
          tunnel: w3472 -> [_ w3522]
          tunnel: [w3496 w3519] -> w3470
          tunnel: w3469 -> [_ w3500]
          tunnel: w3458 -> [_ w3507]
          tunnel: w3464 -> [_ w3505]
          tunnel: w3456 -> [_ w3501]
          tunnel: w3455 -> [_ w3502]
          frame False {
          }
          frame True {
            w3513 = u32 0 ("X-offset IN")
            n2420 = call "DMR_GetImageRequestBufferData.vi"("driver handle IN"=w3523, "request number IN"=w3522) -> ("width OUT"=w3512:i32, "height OUT"=w3511:i32, "driver handle OUT"=w3518:i32, "request number OUT"=w3517:i32, "bytes per pixel OUT"=w3514:i32)  [unwired: 13 out]
            n2421 = call "DMR_GetImageRequestBufferImageData.vi"("driver handle IN"=w3518, "request number IN"=w3517, "bytes per pixel IN"=w3514, "X-offset IN"=w3513, "Y-offset IN"=w3513, "height IN"=w3511, "width IN"=w3512) -> ("driver handle OUT"=w3516:u32, "request number OUT"=w3515:u32, "image OUT"=w3508:u32[][])  [unwired: 10 out]
            n2422 = call "DMR_ImageRequestUnlock.vi"("request number IN"=w3515, "driver handle IN"=w3516) -> ("driver handle OUT"=w3521:i32)  [unwired: 1 in, 2 out]
            n2423 = case shown="True" "Averaging" {
              tunnel: w3508 -> [w3564 w3569]
              tunnel: [w3564 w3568] -> w3504
              tunnel: w3507 -> [_ w3566]
              frame False {
              }
              frame True {
                (unwired) 1
                w3574 = 1
                n2424 = feedback #2(w3566) -> (w3565:u32[][])
                n2425 = Add(x=w3569, y=w3565) -> (x+y=w3570:u32[][])
                n2426 = Select(t=w3566, s="Reset Averaging", f=w3570) -> (s? t:f=w3572:u32[][])
                n2427 = feedback-in #2(w3572) -> ()
                n2428 = feedback #3(w3574) -> (w3567:i32)
                n2429 = Divide(x=w3570, y=w3567) -> (x/y=w3571:dbl[][])
                n2430 = Increment(x=w3567) -> (x+1=w3575:i32)
                n2431 = To Unsigned Long Integer(number=w3571) -> (unsigned 32bit integer=w3568:u32[][])
                n2432 = Select(t=w3574, s="Reset Averaging", f=w3575) -> (s? t:f=w3573:i32)
                n2433 = feedback-in #3(w3573) -> ()
              }
            }
            n2434 = call "DMR_ImageRequestSingle.vi"("request control IN"=0, "driver handle IN"=w3521) -> ("driver handle OUT"=w3519:i32)  [unwired: 3 out]
            n2435 = disable-structure shown="Disabled" {
              disable-tunnel: w3504 -> [w3541 _]
              disable-tunnel: w3501 -> [w3540 _]
              frame Disabled {
                n2436 = To Double Precision Float(number=w3541) -> (double precision float=w3539:dbl[][])
                n2437 = In Range and Coerce(upper limit="Intensity Upper", x=w3539, lower limit="Intensity Lower") -> (coerced(x)=w3538:dbl[][])  [unwired: 1 out]
                n2438 = Subtract(x="Intensity Upper", y="Intensity Lower") -> (x-y=w3535:dbl)
                n2439 = Subtract(x=w3538, y="Intensity Lower") -> (x-y=w3536:dbl[][])
                n2440 = Divide(x=w3536, y=w3535) -> (x/y=w3537:dbl[][])
                n2441 = Multiply(x=255.0, y=w3537) -> (x*y=w3533:dbl[][])
                n2442 = To Unsigned Byte Integer(number=w3533) -> (unsigned 8bit integer=w3542:u8[][])
                n2443 = call "IMAQ ArrayToImage"("Image Pixels (U8)"=w3542, "Image"=w3540) -> ("Image Out"=w3529:T2)  [unwired: 4 in, 5 out]
                n2444 = First Call?() -> (First Call?: T/F=w3530:bool)
                n2445 = case shown="True" w3530 {
                  tunnel: w3529 -> [w3543 w3554]
                  frame False {
                    n2446 = flat-sequence {
                      tunnel: w3543 -> [w3549]
                      frame #0 {
                        w3546 = FALSE ("Get/Set Status? (Set)")
                        w3545 = 0 ("Window Number (0...15)")
                        n2447 = call "IMAQ WindSize"("Get/Set Status? (Set)"=w3546, "Window Number"=w3545) -> ("Width & Height out"=→"Window Size":cluster{"Width":i32, "Height":i32})  [unwired: 4 in, 2 out]
                        n2448 = call "IMAQ WindMove"("Window Number (0...15)"=w3545, "Get/Set Status? (Set)"=w3546) -> ("Coordinates (screen)"=→"Window Position":cluster{"X Position":i32, "Y Position":i32})  [unwired: 3 in, 1 out]
                        n2449 = call "IMAQ WindDraw"("Resize to Image Size? (Y)"=FALSE, "Window Number (0...15)"=w3545, "Image"=w3549) -> ()  [unwired: 7 in, 2 out]
                      }
                      frame #1 {
                        n2450 = call "IMAQ WindZoom 2"("Center Point"="Center Point", "Zoom to Fit? (False)"=FALSE, "Zoom Factor"="Zoom Factor") -> ()  [unwired: 5 in, 4 out]
                      }
                    }
                  }
                  frame True {
                    n2451 = flat-sequence {
                      tunnel: w3554 -> [w3557]
                      tunnel: [w3555] -> w3553
                      tunnel: w3553 -> [w3559]
                      frame #0 {
                        w3556 = TRUE ("Resize to Image Size? (Y)")
                        w3555 = 0 ("Window Number (0...15)")
                        n2452 = call "IMAQ WindNonTearing"("Window Number"=w3555, "NonTearing? (True)"=w3556) -> ()  [unwired: 8 in, 2 out]
                        n2453 = call "IMAQ WindDraw"("Resize to Image Size? (Y)"=w3556, "Window Number (0...15)"=w3555, "Image"=w3557) -> ()  [unwired: 7 in, 2 out]
                      }
                      frame #1 {
                        n2454 = call "IMAQ WindSize"("Scrollbars? (N)"=FALSE, "Width & Height"="Initial Window Size", "Window Number"=w3559) -> ()  [unwired: 3 in, 3 out]
                        n2455 = call "IMAQ WindMove"("Window Number (0...15)"=w3559, "Coordinates (screen)"="Initial Window Position") -> ()  [unwired: 3 in, 2 out]
                      }
                    }
                  }
                }
              }
              frame Enabled {
              }
            }
            n2456 = To Unsigned Byte Integer(number=w3504) -> (unsigned 8bit integer=w3503:u8[][])
            n2457 = call "IMAQ ArrayToImage"("Image Pixels (U8)"=w3503, "Image"=w3500) -> ("Image Out"=w3498:T2)  [unwired: 4 in, 5 out]
            n2458 = case shown="True" "Save Video" {
              tunnel: w3505 -> [_ w3563]
              tunnel: w3498 -> [_ w3562]
              frame False {
              }
              frame True {
                n2459 = call "IMAQ AVI Write Frame"("Image"=w3562, "Avi Refnum"=w3563) -> ()  [unwired: 2 in, 8 out]
              }
            }
            n2460 = case shown="True" "Save Image" {
              tunnel: w3503 -> [_ w3578]
              tunnel: w3502 -> [_ w3577]
              frame False {
              }
              frame True {
                n2461 = call <vilib>:"Flatten Pixmap.vi"("colors"=w3577, "8-bit pixmap"=w3578) -> ("image data"=w3584:T40)  [unwired: 4 in, 5 out]
                n2462 = call "Create new save file.vi"("Insert"="video_frame_" ("string"), "Ext"=".bmp" ("string"), "Index In"="Image Index") -> ("Path Out"=w3580:path, "Index Out"=w3585:dbl)
                n2463 = Increment(x=w3585) -> (x+1=w3579:dbl)
                n2464 = local write "Image Index"(w3579) -> ()
                n2465 = call <vilib>:"Write BMP File.vi"("image data"=w3584, "path to BMP file"=w3580) -> ()  [unwired: 1 in, 9 out]
              }
            }
            n2466 = case shown="True" "Target" {
              tunnel: w3498 -> [w3524 w3528]
              tunnel: [w3524 w3526] -> w3497
              frame False {
              }
              frame True {
                n2467 = local read "Target coordinates"() -> (w3525:cluster{"X1":dbl, "Y1":dbl, "X2":dbl, "Y2":dbl})
                n2468 = call "IMAQ Overlay Oval"("Color"=u32 16711680, "Bounding Rectangle"=w3525, "Image"=w3528) -> ("Image Out"=w3526:T2)  [unwired: 7 in, 1 out]
              }
            }
            "Primary Video Display" <- w3497
          }
        }
        n2469 = node-c288(w3459) -> ()  [unwired: 1 out]
      }
      n2470 = node-c288(w3443) -> ()  [unwired: 1 out]
      n2471 = call "DMR_CloseDevice2.vi"("driver handle IN"=w3448) -> ()  [unwired: 1 in, 4 out]
    }
    frame #4 {
      n2472 = call "DMR_Close.vi"() -> ()  [unwired: 1 out]
    }
  }
  n2473 = local write "Offset (nm)"(0.0 ("Offset (nm)")) -> ()
  n2474 = local write "Bead Mean (nm)"(0.0 ("Bead Mean (nm)")) -> ()
  n2475 = local write "Total Volume\nFlowed P1 (uL)"(w45) -> ()
  n2476 = local write "Total Volume\nFlowed Samp (uL)"(w45) -> ()
  n2477 = local write "Total Volume\nFlowed P3 (uL)"(w45) -> ()
  n2478 = node-c288(i64 1 ("Period"), 1 ("Processor")) -> (w217:T26)  [unwired: 2 out]
  n2479 = timed-loop "Acquire Data" {
    tunnel: w51 -> [w3892]
    tunnel: w98 -> [w3891]
    tunnel: [w3921] -> w309
    tunnel: [w3916] -> w307
    timing: w217 -> [_]
    timing-out: [_] -> w216
    tunnel: w116 -> [w3748]
    stop <- "Stop All" stop-if-true
    w3672 = "Initialize"
    w3738 = "NI_ChannelName" ("name")
    # "I think that the conversion\nfrom 'wiggle amp' to nm\nis 0.277 nm/input. So, 1000\nfor an input is 277 nm."
    n2480 = node-c288() -> ()  [unwired: 2 out]
    n2481 = First Call?() -> (First Call?: T/F=w3707:bool)
    n2482 = Or(x="Reset", y=w3707) -> (x .or. y?=w3708:bool)
    n2483 = local read "Flushing P1"() -> (w3627:bool)
    n2484 = case "Reset data stream" shown="True" w3708 {
      tunnel: w3892 -> [w4957 w4965]
      tunnel: w3891 -> [w4956 w4964]
      tunnel: [w4957 w4959] -> w3620
      tunnel: [w4956 w4958] -> w3887
      frame False {
      }
      frame True {
        w4962 = TRUE ("AI to FIFO")
        n2485 = local write "Overflow (data lost)"(FALSE ("Overflow (data lost)")) -> ()
        n2486 = call "reset FPGA DMA.vi"("error in"=w4964, "FPGA VI Reference In"=w4965) -> ("error out"=w4960:errorcluster, "FPGA VI Reference Out"=w4961:T22)
        n2487 = xnode "Read/Write Control"("FPGA VI Reference In"=w4961, "error in"=w4960, "AI to FIFO"=w4962, "APD to FIFO"=w4962) -> ("FPGA VI Reference Out"=w4959:T22, "error out"=w4958:errorcluster)
      }
    }
    n2488 = case shown="True" w3627 {
      frame False {
      }
      frame True {
        n2489 = local read "Flush rate (uL/m) P1"() -> (w3992:dbl)
        n2490 = local read "HP1 Flush Time (s)"() -> (w3998:dbl)
        n2491 = local read "DMA Update Period (s)"() -> (w3985:dbl)
        n2492 = Divide(x=w3992, y=60.0) -> (x/y=w3984:dbl)
        n2493 = feedback #4(0.0) -> (w3987:dbl)
        n2494 = Divide(x=w3998, y=w3985) -> (x/y=w3990:dbl)
        n2495 = feedback #5(0) -> (w3996:i32)
        n2496 = Increment(x=w3996) -> (x+1=w3989:i32)
        n2497 = Multiply(x=w3985, y=w3984) -> (x*y=w3983:dbl)
        n2498 = Greater?(x=w3989, y=w3990) -> (0:w3995:bool)
        n2499 = Compound Arithmetic op=MULTIPLY(w3985, w3989, w3984) -> (→"P1 Flush Volume (uL)":dbl)
        n2500 = Divide(x=w3989, y=w3990) -> (x/y=→"P1 Flushing Bar":dbl)
        n2501 = Add(x=w3983, y=w3987) -> (x+y=w3986:dbl)
        "Total Volume\nFlowed P1 (uL)" <- w3986
        n2502 = feedback-in #4(w3986) -> ()
        n2503 = case shown="True" w3995 {
          tunnel: w3989 -> [w3999 _]
          tunnel: [w3999 0] -> w3994
          frame False {
          }
          frame True {
            w4000 = FALSE ("Flushing P1")
            n2504 = local write "Inject Pump 1"(w4000) -> ()
            n2505 = local write "Flushing P1"(w4000) -> ()
            n2506 = property on="Clear Volume P1" class="Bool (strict)"("Val(Sgnl)"=TRUE ("Value (Signaling)")) -> ()  [unwired: 2 in, 2 out]
          }
        }
        n2507 = feedback-in #5(w3994) -> ()
      }
    }
    n2508 = Or(x="Start AOD Scan", y="Trap Raster Scan") -> (x .or. y?=w3846:bool)
    n2509 = case "Start AOM raster scan" shown="True" w3846 {
      tunnel: w3620 -> [w4807 w4817]
      tunnel: w3887 -> [w4806 w4816]
      tunnel: [w4807 w4810] -> w3612
      tunnel: [w4806 w4809] -> w3886
      frame False {
      }
      frame True {
        n2510 = case shown="True" "Restart DMA? (AOD)" {
          tunnel: [w4855 w4857] -> w4811
          tunnel: [w4854 w4856] -> w4812
          tunnel: w4817 -> [w4855 w4859]
          tunnel: w4816 -> [w4854 w4858]
          frame False {
          }
          frame True {
            n2511 = local write "Overflow (data lost)"(FALSE ("Overflow (data lost)")) -> ()
            n2512 = call "reset FPGA DMA.vi"("error in"=w4858, "FPGA VI Reference In"=w4859) -> ("error out"=w4856:errorcluster, "FPGA VI Reference Out"=w4857:T22)
          }
        }
        n2513 = local write "Trap Raster Scan"(FALSE ("Trap Raster Scan")) -> ()
        n2514 = case shown="False" "Move MCL Also?" {
          tunnel: w4812 -> [w4821 w4849]
          tunnel: w4811 -> [w4822 w4850]
          tunnel: [w4820 w4853] -> w4810
          tunnel: [w4819 w4852] -> w4809
          frame False {
            w4818 = TRUE ("AI to FIFO")
            n2515 = xnode "Read/Write Control"("FPGA VI Reference In"=w4822, "error in"=w4821, "AI to FIFO"=w4818, "APD to FIFO"=w4818, "Start scan"=w4818) -> ("FPGA VI Reference Out"=w4820:T22, "error out"=w4819:errorcluster)
          }
          frame True {
            w4846 = FALSE ("1D or 2D Scan?")
            w4851 = TRUE ("AI to FIFO")
            # "Count for MCL loop"